vi "Decimate.vi"() -> (3 "2-Stage Decimation: Octaves 2-8":T1[](array[typedef])=[{"VSignalRMS"=3.569254560184283, "VNoiseRMS"=0.0015456498604675313, "SNR(dB)"=67.26932808076202, "NumBits"=10.881948186173094, "SNRFS(dB)"=67.18687774967906, "NumBitsFS"=10.868252117886886}, {"VSignalRMS"=3.569302135994948, "VNoiseRMS"=0.0015758831325008, "SNR(dB)"=67.1011860962303, "NumBits"=10.854017623958521, "SNRFS(dB)"=67.01861998873524, "NumBitsFS"=10.840302323710173}, {"VSignalRMS"=3.569179527030871, "VNoiseRMS"=0.0015457687304173328, "SNR(dB)"=67.26847751090318, "NumBits"=10.881806895498867, "SNRFS(dB)"=67.18620977720272, "NumBitsFS"=10.868141159003773}, {"VSignalRMS"=3.569284052806068, "VNoiseRMS"=0.0015488080787911924, "SNR(dB)"=67.25167012588723, "NumBits"=10.879014971077613, "SNRFS(dB)"=67.16914802390777, "NumBitsFS"=10.865306980715575}, {"VSignalRMS"=3.569278212241904, "VNoiseRMS"=0.0015445316735475394, "SNR(dB)"=67.27567164377996, "NumBits"=10.883001934182717, "SNRFS(dB)"=67.1931637548854, "NumBitsFS"=10.86929630479824}, {"VSignalRMS"=3.5692565348659597, "VNoiseRMS"=0.0010534504316992595, "SNR(dB)"=70.59927315773149, "NumBits"=11.435095208925496, "SNRFS(dB)"=70.51681802120187, "NumBitsFS"=11.421398342392337}, {"VSignalRMS"=3.569299509403375, "VNoiseRMS"=0.0007252888840803322, "SNR(dB)"=73.84143941716077, "NumBits"=11.97366103275096, "SNRFS(dB)"=73.75887970147343, "NumBitsFS"=11.95994679426469}, {"VSignalRMS"=3.569262170230891, "VNoiseRMS"=0.0004828117383160924, "SNR(dB)"=77.3760125744556, "NumBits"=12.560799430972692, "SNRFS(dB)"=77.29354372411225, "NumBitsFS"=12.547100286397384}, {"VSignalRMS"=3.56927087447335, "VNoiseRMS"=0.00037148318496641716, "SNR(dB)"=79.65280695478424, "NumBits"=12.93900447753891, "SNRFS(dB)"=79.57031692247287, "NumBitsFS"=12.925301814364264}] {"SNRFS(dB)" format="%_3p"; "NumBitsFS" format="%.1f"; "NumBits" format="%.1f"; "SNR(dB)" format="%_3p"; "VNoiseRMS" format="%#_3p"; "VSignalRMS" format="%#_3p"}, 11 "Input":waveform(dbl)[](graph)=[{"t0"=timestamp(0 s since 1904-01-01), "dt"=1e-07, "Y"=array[200000 elements]}, {"t0"=timestamp(0 s since 1904-01-01), "dt"=1e-07, "Y"=array[200000 elements]}] caption="Histogram")   [LabVIEW 2019] (continued)
-89.8010347026674, -91.03397353010905, -93.05880817130885, -93.86569223660774, -93.37353857073721, -94.99416885665839, -99.05596611693173, -107.36497646738917, -102.6044915270977, -96.19397229786782, -96.1597538289888, -102.83527542224925, -97.10995031748254, -93.13768460557588, -93.6872108649518, -96.88332215210443, -91.8911442399971, -88.87814381179629, -89.52765316051676, -90.61283401268693, -88.61347146837466, -86.64246320759895, -87.20248076787445, -89.71664016321188, -92.17437436351524, -96.52818073700101, -102.89028350758038, -95.51571015309541, -90.29404249884288, -88.78950020057246, -90.05141478281257, -93.14256393856814, -96.4338383803238, -98.1272334355839, -98.38148782151309, -98.52874806510161, -97.52896129220633, -93.04723881975156, -88.27184928640632, -85.88377796724602, -85.65268972364586, -86.59982678770758, -88.4789647414978, -91.7805915661704, -97.07047803294813, -107.73747761660528, -98.60351784227328, -93.52998614692484, -93.33290182993952, -96.85531600078095, -96.37376134080165, -90.69117698738063, -88.14576852093532, -88.25747447952166, -90.45082399151303, -96.41863707301175, -101.4196021122521, -93.96770566579788, -93.58811415156053, -96.07316515859912, -95.5343037432213, -96.69546499020845, -103.82710137540842, -91.0904529950192, -86.73242770513536, -86.46505143994031, -88.73991396184971, -92.4473353636468, -95.59367731654704, -91.48494027019697, -87.58229561240861, -85.91683271877996, -85.80490261027448, -86.60468865692945, -88.2671187787114, -91.43151609166779, -96.08162874738761, -97.96724691276759, -97.11638853174621, -99.15289822897408, -123.93308240573889, -100.23264801665928, -97.93670882000998, -101.99411747199824, -108.2661715906857, -95.01879672304669, -93.09344762172648, -97.96569428999419, -103.31348133169591, -94.56331004427977, -91.27392525391764, -89.86929621291289, -90.5326639141475, -93.30981422202001, -94.64433988957715, -93.81030718221622, -92.11600765997169, -90.47514602466164, -91.6034286338698, -91.52808955554679, -88.72387392453297, -90.22769969249696, -101.22756810629461, -93.02935870824089, -88.75723657607486, -89.07116344980949, -91.5022695405016, -92.33189422244578, -92.15231627049769, -96.429614181429, -97.34230671596741, -90.58396100985783, -87.14766416331051, -85.85891058335328, -86.31876359404814, -89.10677082541883, -97.31293864995898, -101.61260941340501, -96.67024962948099, -95.7803144954672, -92.23018395709333, -91.92293467829664, -95.19175145715253, -100.08921092086965, -100.05799390116158, -99.02803629195597, -109.28207521152451, -96.6021839187509, -90.38957395013965, -90.28504566646042, -93.17850262164265, -93.71200868183445, -97.4244039887505, -97.21740806348627, -89.14256467259328, -87.44588011755873, -90.97086244268247, -109.87431813081962, -96.94460754937701, -93.86113811879602, -91.86280043107433, -91.70994113858619, -92.89616081483194, -90.50118183916814, -90.18614880163818, -94.52151436094952, -100.73253124580648, -99.8220360349123, -100.29830396810995, -107.49078067194083, -94.01601739016263, -91.24863884043859, -94.98674357343711, -104.57651242950692, -99.85629224470014, -108.93064387422969, -93.53962952692434, -90.00240167674333, -90.68494946709862, -93.29637143102863, -94.60776650516321, -92.67968715579968, -90.33204021940706, -90.55631207399716, -92.43577805509032, -89.15503146181992, -86.30010955844271, -86.83979289314496, -89.48485493821893, -88.96405338383319, -87.52421931179818, -87.60531529349264, -88.6702529441048, -90.89292417707969, -95.88440563526038, -96.46881508553417, -91.06541812352924, -91.35314766368683, -99.08109799743801, -93.35876385631522, -88.11981688709662, -86.17097485203567, -85.52792069986612, -86.04182686687071, -88.51643246854445, -95.16445751359271, -100.73666271200408, -92.65818704084369, -93.12039396890881, -101.9336312438025, -96.2875533856691, -92.86539060044441, -92.38339167479018, -91.61776239409015, -89.00733167601517, -86.75068814616338, -86.11927241760986, -86.43308873694038, -86.39221303948099, -86.66783030203213, -88.67265978744017, -92.24294564543717, -95.12190286714484, -95.27152864373058, -93.34130562149033, -89.80175424374963, -87.41382180737244, -88.04182405274452, -91.15829518615249, -94.8596085864744, -99.07780397052106, -95.01095310320474, -91.45492540453984, -88.85659471003605, -88.09703705871516, -91.14850708600869, -102.48113857609522, -95.20951614488438, -90.76054140267786, -89.82778110342488, -90.66593638186606, -91.75679507239694, -90.08765062811106, -88.65512843108004, -89.86771840104606, -93.11899129528413, -95.07880434483995, -93.66805564380138, -91.82378563741104, -91.42798403486283, -93.33242715271743, -94.46541343567961, -95.10490793802889, -95.23778068069765, -89.91147243285879, -84.72844146564022, -83.12294491520029, -84.9529908072355, -89.20201404077906, -93.39646902993033, -90.84293632205467, -88.26483479024421, -87.52146927444474, -88.27666880088361, -89.15187738597957, -90.11954936247787, -94.16844824268043, -107.89828675933434, -92.96950334185829, -88.238044809099, -86.53155469309384, -86.00724711483737, -85.84166713830888, -86.34560567244318, -88.05752912180658, -89.45912806461533, -89.2035558192775, -90.26794762923997, -94.61492559085042, -93.47913197993867, -89.68023195055093, -88.5844007239764, -88.16209645670403, -87.69248229261242, -88.19926215150255, -89.03813165364234, -88.23806114711809, -86.06271848210922, -84.55338844577818, -84.60581192467787, -85.1077884922066, -84.87483822256023, -86.29645607493103, -92.06433822589182, -107.45719303754848, -112.34185245802342, -100.81236537855537, -95.98023535529101, -97.06022523776083, -108.91939984092842, -104.58355826222842, -105.28926347697224, -98.10962881250319, -91.97176200903287, -90.1266388214861, -90.67818031849367, -92.85563489938073, -93.76500929039366, -91.5852495688892, -91.19048588685934, -93.62384628504867, -93.7795356927555, -91.19750841744859, -90.74358943616139, -93.00542929634658, -94.3681235267732, -90.8623272907447, -90.01485035029057, -92.52070202183269, -98.91906043598311, -102.5897642561925, -99.82530029415895, -102.20958845474463, -107.13921947376252, -107.01853509868056, -110.28556884145588, -103.44422077868307, -94.7252960700585, -91.45806458223853, -93.42525832838932, -97.31725729774752, -95.44946115186846, -94.8595760042268, -94.1498831531218, -93.04365469327082, -92.03054869023626, -91.77414183713913, -94.41138276683348, -98.48171674510718, -95.05341322220156, -94.82148351748654, -97.08324798828943, -92.96605208041271, -89.34070749513245, -88.29777010929871, -88.30288027606483, -89.48962380854178, -93.82108906158335, -96.51961583222484, -95.21010881511009, -100.42640215279664, -108.00389623621597, -100.31346689277512, -98.771133498524, -96.92097352108053, -96.52772982975304, -103.85461800825347, -98.4364859896675, -96.75691862450641, -99.93868436121357, -101.0553868817555, -101.80612831811997, -102.32522849853484, -114.90329875071347, -97.84170076615057, -90.72356335005702, -88.75686077967089, -90.93220347773621, -100.31068639097393, -92.6918740853231, -87.47727509271918, -86.40638848521573, -87.31674769566013, -88.8718261906175, -90.84717782219451, -96.14111518295532, -112.7387467405839, -96.80330128832384, -94.49443144832229, -93.1187694720117, -94.09577295380575, -97.84347233566405, -98.83196403782361, -102.66702576290031, -102.06740338682923, -96.98779181032735, -95.60219419087134, -96.27567410728503, -97.38558620235028, -101.70178505678969, -105.17955779424086, -92.53192910654218, -88.81788220476069, -88.95711618627857, -92.57722780091505, -95.93532470547275, -94.91138856116832, -94.10808424076805, -91.07784296453154, -90.66312583820053, -94.83055022969745, -93.45801693898999, -88.36453147845204, -86.51183079184831, -86.25944696127009, -87.45497047294643, -89.96042118208382, -92.69280919745722, -95.17516080722282, -97.2545095704103, -108.19727080658595, -94.98874557277178, -88.7096850874034, -88.29851760651509, -92.97093470402908, -109.47313678444067, -92.15693004585063, -89.54380160860075, -91.20532066404374, -94.01507769477956, -98.32922344795767, -115.87223636278607, -104.99730428404263, -97.90500783504449, -93.52723553984637, -92.68564560569936, -95.29601374056632, -98.60820212308043, -95.8632487136141, -95.62504147674952, -96.80363703429067, -93.03623657868951, -90.52579360619532, -90.264401776805, -92.92037685812984, -103.55931238637702, -100.10371390759235, -97.64269926597996, -106.70160125220791, -103.46147653543306, -104.92381444474447, -97.66898940024639, -98.1207217224727, -102.97619867092016, -98.71215110846583, -97.0432854793485, -99.16590358458605, -108.7063174536745, -100.82749343291766, -96.03893851051149, -91.58971668752456, -89.61426914396401, -90.35560864138453, -92.20810749474501, -92.89100216232576, -93.49681684033557, -99.76551973814325, -97.0799906106162, -90.31362726389034, -88.57325340330499, -88.96730438665082, -90.26248640164394, -90.52895855114714, -90.20987348700926, -93.00267887063752, -94.17584736186727, -88.81040704570617, -86.93952112623633, -87.9056288932579, -91.98566538263984, -100.15858921606016, -103.76052918019197, -96.71723266703998, -93.03577725134335, -94.72780454891021, -103.01451117711142, -97.6699107089091, -96.01913455617363, -110.1206312200923, -91.92605804348743, -88.00078024686586, -87.8880681034834, -87.30056231006418, -85.83303495316628, -85.85418846348472, -87.7821464251187, -90.2758402998394, -90.88533878280161, -90.8459208229611, -93.28890303633764, -96.45506943175144, -93.9657279319056, -95.14678514742427, -103.76092783519839, -93.51369734169444, -89.15496358093812, -88.94760221872505, -93.21836724942621, -102.70177680497022, -94.3088663314495, -94.4492283335647, -107.54669077263702, -95.02325691171124, -89.94809305281855, -88.76442278570764, -90.15843384117183, -94.18927428924788, -103.5607343640872, -104.71985453910293, -97.44689724688605, -96.66538549864534, -92.99791884731977, -88.91345920971567, -88.78289126806351, -93.20237581867212, -99.61032143489241, -98.03939989557719, -93.0026775167182, -91.81883719675187, -93.16528083057023, -91.99657831882547, -90.82862397733015, -90.35913544748666, -88.27997681101144, -87.06043651234096, -90.01623158825575, -98.26998906374854, -98.87182053703206, -97.96821523251893, -100.72261242087296, -103.61735109062678, -100.97137969331385, -96.99686450208753, -99.11583654269441, -96.80933076136141, -89.94358046453371, -90.5589653328009, -98.05169889385459, -93.71424181113524, -90.43633068673337, -92.57816106624148, -103.50808505873314, -100.01204811846273, -93.81345468138845, -92.31007899066856, -92.41740595409402, -92.79570377679568, -93.82486981119445, -98.31226033178805, -101.74612278185292, -94.3497825868709, -90.69857292290774, -88.78277526094769, -88.77097805601, -89.94284365081724, -90.70689274098581, -91.5148685235682, -93.14799332791, -94.81640407745275, -98.81943039379316, -106.08095876700384, -95.18999798662253, -92.4142146852307, -92.57021663897197, -92.66199047832845, -91.92099703946455, -90.03706209531208, -87.38587815679551, -85.87225930549337, -86.2255296819672, -88.28775142723944, -93.27505872274777, -115.99751912628982, -92.53915821293742, -87.9207035231365, -85.55641230589154, -84.94877133314154, -86.88955282712729, -93.96785309236557, -94.0289793243198, -87.4272553612049, -87.29762396991052, -92.30440971489529, -120.21878514409582, -95.00976512147977, -91.31588049120478, -90.56898331734459, -90.77858748375854, -91.89648836362517, -96.29348753218406, -100.93249278623325, -97.32178285939624, -98.62014208276622, -100.48562472201668, -97.33369690760833, -95.00343910264645, -95.69979646246864, -98.74130162362789, -100.27898936972626, -94.9378052586386, -90.20931572958756, -88.53058670603681, -88.27380374992417, -87.20092602666031, -86.05931266172865, -87.22653057818638, -91.39673283963971, -95.38223908175, -95.96072073705783, -99.42329566628243, -98.34654372546375, -93.4993314587484, -92.89016890488827, -92.02184448181553, -92.17619172419795, -96.26933765840184, -98.18453485909882, -93.66052810216247, -90.8323686849731, -90.36431799650393, -91.97615119961696, -96.46500758909855, -94.96914243908718, -91.01807463861238, -91.2779918513813, -92.96017533514774, -95.42849867438704, -101.77004213826638, -105.27901395308567, -99.56242545898206, -97.90225814801475, -101.28031650242258, -96.1015978589149, -93.34246627165528, -93.70559141177273, -94.20889705360737, -93.81582595663994, -94.06324580025588, -95.19473180113226, -92.86573512497009, -89.18354883248035, -88.20359411470437, -89.89806767859326, -91.91816476953262, -89.77231066774974, -88.18071979990691, -88.0280893835839, -88.04423231379133, -88.80392977533683, -91.19824097961524, -98.58922742068387, -95.30068248468645, -90.02940744460808, -89.92923732451595, -96.44564808729093, -99.96939540191892, -91.78821600214482, -91.34013881425585, -91.68182786268892, -92.75576407614253, -97.60096039215023, -110.79584639656908, -100.7398169767965, -98.90169971973356, -96.98475068395564, -91.24777218925851, -87.14164582650936, -85.07841513945877, -85.26972079412609, -87.22392671417005, -88.00822550141241, -87.76027181453824, -89.58415902951826, -92.4920968244888, -91.52877820490346, -90.95171438597555, -95.41394558528829, -107.52016977965116, -93.55378221755299, -93.09841424146704, -96.03020240280674, -92.62019862066694, -90.37102864174886, -90.32746097852643, -91.64498883121686, -90.32100090650229, -87.3315532070872, -85.03676944258837, -83.85985926521577, -84.73848912491917, -87.6784018437611, -90.04115270468093, -91.25387893030472, -93.23095692661319, -95.25231864597927, -97.66363332944596, -102.77464914802627, -101.15895720449821, -99.62005914650605, -102.63735241934043, -104.85039530539925, -101.25579402001435, -99.77764723417644, -101.57938969988805, -99.1058053458501, -96.33289113064549, -94.41799875122697, -93.49242925347608, -94.50404330381863, -96.76817317436303, -93.93672457673864, -91.29474684489637, -93.26842869447049, -102.42081187230232, -103.08983670436645, -109.52250784041115, -97.2726279572302, -89.96149106309333, -88.13167591404391, -89.17627713478488, -90.81731028389734, -89.69598642936998, -89.38981783502201, -89.50603404532913, -88.89585545757966, -89.56629637073901, -90.96578900098268, -91.22149297466228, -91.3785919844561, -93.15397967041592, -94.4901683525819, -92.7368020668827, -92.14949353336037, -94.95758584517533, -103.64001941535494, -102.27201854610108, -94.06232889812578, -92.93522322915264, -95.7335577608483, -97.6724118748942, -93.40509883173105, -93.66687115451643, -101.02764174706243, -99.12707487021106, -94.48016277568419, -94.67470865634454, -98.42431273446714, -103.24880029559685, -99.90925994581126, -95.15695525887934, -93.41579558721341, -94.67409325043697, -95.82278490747215, -94.14142963683659, -93.06397710154005, -94.67664396404518, -98.33033807601927, -93.38609170228307, -90.11276515968119, -88.90838552954386, -87.56195891881562, -86.61620485564832, -87.44524687073933, -90.90537825376526, -96.54713542070294, -93.39343846176016, -91.65569563103823, -92.14374689709948, -93.25103368600128, -97.10001809735326, -92.95120769052104, -86.90162204337808, -85.96113002826127, -89.22843563290024, -99.98215601142925, -93.87545654951096, -88.52698412964402, -90.35913274669417, -100.91895124333183, -92.48828884459081, -89.52817506852307, -90.85947850957027, -94.57527777304777, -99.5269326990987, -99.60633181869059, -95.72628145429307, -95.03394942536164, -94.1117243729267, -92.45824814083, -93.20733286443966, -94.21187595555205, -91.14499167368595, -88.47301855464184, -87.65697415447646, -89.3491095696534, -93.80345111261569, -99.68008971154478, -100.12908406450812, -94.31594799973227, -92.32494145325448, -93.75927524111154, -93.24162555187677, -91.83340564056253, -91.39583615477781, -92.9927938979383, -99.32988111167916, -102.36851511008263, -94.21226623786877, -89.50102510569984, -87.52005746489233, -88.47429326228288, -94.18062027460594, -97.08519622981159, -88.44622877710566, -87.17483083286665, -90.53412682553531, -98.80032159988284, -112.0139605538499, -114.73822729493698, -108.47097394029929, -107.04801965347384, -103.79117249163477, -93.69620484132517, -90.20414443914342, -90.93394829658737, -93.89847212895639, -95.25161152513147, -94.67463116505695, -94.65303698780667, -96.52871287518005, -103.59167379262703, -97.3093661652524, -93.13057204576113, -93.48726944940366, -96.97938502988173, -100.05124973201501, -94.39188624348108, -91.47606085909311, -92.9112596329322, -96.52898769576653, -95.93029258632751, -91.36739129728717, -90.64709732022601, -92.33074646702256, -93.12266929064732, -92.710435012283, -93.66993194171718, -96.66266310132755, -101.86758330767772, -102.0049247869093, -97.6442479953907, -95.68999770184644, -95.70255601030347, -91.85350103951814, -88.66409645137753, -88.97899246700999, -92.47972679191342, -94.19740594455185, -89.79975447682834, -88.06347092046212, -89.50744525042023, -94.90319594188456, -102.73396352972853, -97.78022699866135, -96.41875055142742, -97.61374856205884, -101.14594314754896, -91.07819652365637, -86.20151492090294, -84.43580987646789, -84.40343321539262, -85.4512275674312, -86.95812160502341, -87.38158628291737, -86.92750011319069, -87.59641317432796, -90.8808100008769, -98.66278213466741, -92.07358739303535, -86.66872385575152, -84.81103040399233, -85.15216430890109, -86.3701227119982, -86.99273267548816, -87.56139630381969, -89.59164806271204, -93.90931125716035, -94.7747826643407, -90.81810446669623, -88.25377581259738, -86.89687153931219, -87.00420294319926, -89.66919632785404, -97.97802217885085, -101.1543714645282, -92.01004343018782, -88.48812761828798, -86.37140706971644, -85.30861499609067, -85.50676823397659, -87.04715207432281, -89.56919372991476, -91.21639006182731, -90.00710468462273, -87.56326618667731, -85.71087905629356, -85.256302358152, -86.02039260583963, -85.95860793013176, -84.9597151895099, -85.47467902194902, -88.17529871401237, -94.46151142269389, -104.4795994742826, -90.62205386572919, -86.60259576725531, -86.15117934101244, -88.14061646864911, -90.22552942827053, -90.23075884569806, -88.9795464994569, -88.09496890634763, -88.10286347397336, -89.29342654721987, -91.97001454391268, -94.97369664752816, -94.58282592742778, -93.03651295821604, -91.73180808496429, -89.4413987639919, -88.1062492362812, -89.08416681250316, -92.00463005101325, -94.46986101023663, -94.98934726061613, -94.75619871742677, -95.15939521180876, -100.30338510222867, -100.72723563767974, -90.65610684683526, -87.78121672994476, -88.9486698831994, -94.27478448469651, -103.54935817879945, -98.06669656253065, -93.91758818564313, -93.47079131141024, -92.04208725685709, -90.6451361739226, -90.76636107274352, -90.42103213618275, -90.56286879665706, -91.72390699440554, -94.00932025463854, -101.33128658211626, -105.61432288405747, -100.71871174366068, -95.43418166984756, -91.226388311365, -92.05115080560162, -94.90602236858494, -94.7278081014079, -92.50147105725247, -91.73088417004178, -93.99995298481683, -100.77630752561265, -92.24736653451953, -87.34945508143532, -86.32547617096144, -87.72396565284308, -91.61940201299744, -102.83952571655541, -98.57454225038964, -92.11235735605948, -90.82153081888086, -93.22653255311293, -100.57820257707947, -100.71490844146241, -93.27806436638666, -89.81672883858188, -89.43584378033519, -91.49478107995014, -91.23005227675968, -89.87906075424215, -91.22224554955343, -94.36330957997907, -96.57020876047248, -98.47960211136326, -102.60206932430148, -97.85025869384859, -95.62004803407247, -96.82074626938368, -95.36641190186579, -94.62955480252799, -96.56732905283187, -99.78488099782834, -95.54134836047314, -90.85106276396188, -91.53811864957345, -97.35398945483547, -99.53390924269618, -95.50550211172002, -94.24883407244174, -95.15845296283891, -92.52876949052072, -89.18489265592221, -88.3231593450649, -90.21847755944741, -96.28601451043076, -96.42148418004156, -90.0423710177557, -88.35384430411479, -88.45800104614098, -87.39915267866814, -84.9649415862749, -83.05546796952149, -82.53813288647429, -83.62358980677735, -86.64329516486029, -92.49839132920357, -100.96627720063958, -102.03774536659961, -101.55721936960227, -101.4919591633547, -109.49368516118811, -100.54156324375568, -93.1995924271338, -91.95610626225269, -94.54326224475864, -94.45480287553445, -90.63645329465285, -89.06115591026294, -89.13290400541244, -89.03992767460898, -88.35162930135266, -88.46227802743762, -88.71864528174883, -87.14494782239026, -85.75618719388423, -86.7517555817581, -89.70602126044467, -91.9312021642449, -93.10715040857424, -95.09804072655095, -93.67107590708542, -88.79809377890399, -85.4813978604545, -84.97790290229165, -87.26875120136336, -91.81955749355437, -93.97436752534212, -93.17419492057974, -94.72899092677758, -101.50873916930624, -102.42854835344474, -90.93542725599947, -86.91428707756133, -87.10383889824635, -89.09108940684278, -88.4500883642402, -86.62101390069743, -85.92383744773456, -85.91510889390906, -85.89392970945173, -86.18538075642498, -87.06255280982421, -89.6041373377338, -97.37862658290312, -96.5067648178377, -89.45694870912129, -86.72282125077987, -84.7805642597111, -82.9102759515595, -82.19689500929915, -83.06278673741679, -84.61305596458077, -85.57445584067696, -86.0152215595378, -86.49448845038934, -86.21839866020926, -85.33030186000204, -86.20000801703499, -90.11626361376807, -93.71043548054743, -91.20571923212147, -88.34768634049867, -88.05561567210353, -90.11882678795826, -92.79075903663114, -92.53274818890827, -90.15586226108351, -89.7588785406825, -92.51437122484617, -96.88253109308307, -95.01965867485444, -89.4020940322562, -87.36029269867059, -88.40574804749141, -89.39108945249801, -89.2136953159512, -90.0825705642915, -93.5797629864681, -100.02421686821893, -97.37689573314105, -91.15170800268984, -89.62276780794588, -91.81358650078799, -96.1459571696283, -98.78905079920406, -95.90966812857447, -91.0005558312157, -89.42715635616975, -91.23884179011795, -97.4530564846785, -103.85666825119125, -96.25176115537727, -93.62539913970993, -93.03047254411906, -93.6940820406606, -93.61728990851228, -90.37925780092463, -87.38864297445694, -88.18397636144071, -96.3132450903164, -89.02089079629584, -84.41432793280624, -83.65030393991381, -84.44637248702462, -85.87910745894929, -87.96238438851253, -90.95552843255147, -95.23385561565782, -99.98676571010093, -98.25033889671077, -92.9148387998585, -90.76261672348406, -92.44105364838288, -97.36071315590407, -102.36442424446955, -106.64846134350339, -100.6227402487165, -96.18879414360443, -94.50781769211488, -94.24616329879782, -93.08870297958529, -93.04485425173121, -97.00614950521859]} caption="Histogram"
  out "filter information 2":T3={"magnitude H(w)"={"f0"=0.0, "df"=4882.8125, "Mag H(w)"=[0.0, 0.0, 0.0, -0.0, 0.0, 0.0, -0.0, -0.0, -0.0, 0.0, 0.0, 0.0, 0.0, 0.0, 0.0, 0.0, 0.0, -0.0, -0.0, -0.0, -0.0, -0.0, -0.0, -0.0, -0.0, -0.0, -0.0, -0.0, -0.0, -0.0, -0.0, -0.0, 0.0, 0.0, 0.0, 0.0, 0.0, 0.0, 0.0, 0.0, 0.0, 0.0, 0.0, 0.0, 0.0, 0.0, 0.0, 0.0, 0.0, -0.0, -0.0, -0.0, -0.0, -0.0, -0.0, -0.0, -0.0, -0.0, -0.0, -0.0, -0.0, -0.0, -0.0, -0.0, 0.0, 0.0, 0.0, 0.0, 0.0, 0.0, 0.0, 0.0, 0.0, 0.0, 0.0, 0.0, 0.0, 0.0, 0.0, 0.0, 0.0, -0.0, -0.0, -0.0, -0.0, -0.0, -0.0, -0.0, -0.0, -0.0, -0.0, -0.0, -0.0, -0.0, -0.0, -0.0, -0.0, 0.0, 0.0, 0.0, 0.0, 0.0, 0.0, 0.0, 0.0, 0.0, 0.0, 0.0, 0.0, 0.0, 0.0, 0.0, 0.0, -0.0, -0.0, -0.0, -0.0, -0.0, -0.0, -0.0, -0.0, -0.0, -0.0, -0.0, -0.0, -0.0, -0.0, -0.0, 0.0, 0.0, 0.0, 0.0, 0.0, 0.0, 0.0, 0.0, 0.0, 0.0, 0.0, 0.0, 0.0, 0.0, 0.0, 0.0, 0.0, -0.0, -0.0, -0.0, -0.0, -0.0, -0.0, -0.0, -0.0, -0.0, -0.0, -0.0, -0.0, -0.0, -0.0, -0.0, 0.0, 0.0, 0.0, 0.0, 0.0, 0.0, 0.0, 0.0, 0.0, 0.0, 0.0, 0.0, 0.0, 0.0, 0.0, 0.0, 0.0, -0.0, -0.0, -0.0, -0.0, -0.0, -0.0, -0.0, -0.0, -0.0, -0.0, -0.0, -0.0, -0.0, -0.0, -0.0, -0.0, 0.0, 0.0, 0.0, 0.0, 0.0, 0.0, 0.0, 0.0, 0.0, 0.0, 0.0, 0.0, 0.0, 0.0, 0.0, 0.0, -0.0, -0.0, -0.0, -0.0, -0.0, -0.0, -0.0, -0.0, -0.0, -0.0, -0.0, -0.0, -0.0, -0.0, -0.0, -0.0, 0.0, 0.0, 0.0, 0.0, 0.0, 0.0, 0.0, 0.0, 0.0, 0.0, 0.0, 0.0, 0.0, 0.0, 0.0, 0.0, -0.0, -0.0, -0.0, -0.0, -0.0, -0.0, -0.0, -0.0, -0.0, -0.0, -0.0, -0.0, -0.0, -0.0, -0.0, -0.0, 0.0, 0.0, 0.0, 0.0, 0.0, 0.0, 0.0, 0.0, 0.0, 0.0, 0.0, 0.0, 0.0, 0.0, 0.0, 0.0, -0.0, -0.0, -0.0, -0.0, -0.0, -0.0, -0.0, -0.0, -0.0, -0.0, -0.0, -0.0, -0.0, -0.0, -0.0, 0.0, 0.0, 0.0, 0.0, 0.0, 0.0, 0.0, 0.0, 0.0, 0.0, 0.0, 0.0, 0.0, 0.0, 0.0, 0.0, 0.0, -0.0, -0.0, -0.0, -0.0, -0.0, -0.0, -0.0, -0.0, -0.0, -0.0, -0.0, -0.0, -0.0, -0.0, -0.0, 0.0, 0.0, 0.0, 0.0, 0.0, 0.0, 0.0, 0.0, 0.0, 0.0, 0.0, 0.0, 0.0, 0.0, 0.0, 0.0, 0.0, -0.0, -0.0, -0.0, -0.0, -0.0, -0.0, -0.0, -0.0, -0.0, -0.0, -0.0, -0.0, -0.0, -0.0, -0.0, 0.0, 0.0, 0.0, 0.0, 0.0, 0.0, 0.0, 0.0, 0.0, 0.0, 0.0, 0.0, 0.0, 0.0, 0.0, 0.0, 0.0, -0.0, -0.0, -0.0, -0.0, -0.0, -0.0, -0.0, -0.0, -0.0, -0.0, -0.0, -0.0, -0.0, -0.0, -0.0, 0.0, 0.0, 0.0, 0.0, 0.0, 0.0, 0.0, 0.0, 0.0, 0.0, 0.0, 0.0, 0.0, 0.0, 0.0, 0.0, 0.0, -0.0, -0.0, -0.0, -0.0, -0.0, -0.0, -0.0, -0.0, -0.0, -0.0, -0.0, -0.0, -0.0, -0.0, -0.0, 0.0, 0.0, 0.0, 0.0, 0.0, 0.0, 0.0, 0.0, 0.0, 0.0, 0.0, 0.0, 0.0, 0.0, 0.0, 0.0, 0.0, -0.0, -0.0, -0.0, -0.0, -0.0, -0.0, -0.0, -0.0, -0.0, -0.0, -0.0, -0.0, -0.0, -0.0, -0.0, 0.0, 0.0, 0.0, 0.0, 0.0, 0.0, 0.0, 0.0, 0.0, 0.0, 0.0, 0.0, 0.0, 0.0, 0.0, 0.0, 0.0, -0.0, -0.0, -0.0, -0.0, -0.0, -0.0, -0.0, -0.0, -0.0, -0.0, -0.0, -0.0, -0.0, -0.0, -0.0, 0.0, 0.0, 0.0, 0.0, 0.0, 0.0, 0.0, 0.0, 0.0, 0.0, 0.0, 0.0, 0.0, 0.0, 0.0, 0.0, 0.0, -0.0, -0.0, -0.0, -0.0, -0.0, -0.0, -0.0, -0.0, -0.0, -0.0, -0.0, -0.0, -0.0, -0.0, -0.0, 0.0]}, "phase H(w)"={"f0"=0.0, "df"=4882.8125, "Phase H(w)"=[0.0, 0.0, 0.0, -0.0, 0.0, 0.0, -0.0, -0.0, -0.0, 0.0, 0.0, 0.0, 0.0, 0.0, 0.0, 0.0, 0.0, -0.0, -0.0, -0.0, -0.0, -0.0, -0.0, -0.0, -0.0, -0.0, -0.0, -0.0, -0.0, -0.0, -0.0, -0.0, 0.0, 0.0, 0.0, 0.0, 0.0, 0.0, 0.0, 0.0, 0.0, 0.0, 0.0, 0.0, 0.0, 0.0, 0.0, 0.0, 0.0, -0.0, -0.0, -0.0, -0.0, -0.0, -0.0, -0.0, -0.0, -0.0, -0.0, -0.0, -0.0, -0.0, -0.0, -0.0, 0.0, 0.0, 0.0, 0.0, 0.0, 0.0, 0.0, 0.0, 0.0, 0.0, 0.0, 0.0, 0.0, 0.0, 0.0, 0.0, 0.0, -0.0, -0.0, -0.0, -0.0, -0.0, -0.0, -0.0, -0.0, -0.0, -0.0, -0.0, -0.0, -0.0, -0.0, -0.0, -0.0, 0.0, 0.0, 0.0, 0.0, 0.0, 0.0, 0.0, 0.0, 0.0, 0.0, 0.0, 0.0, 0.0, 0.0, 0.0, 0.0, -0.0, -0.0, -0.0, -0.0, -0.0, -0.0, -0.0, -0.0, -0.0, -0.0, -0.0, -0.0, -0.0, -0.0, -0.0, 0.0, 0.0, 0.0, 0.0, 0.0, 0.0, 0.0, 0.0, 0.0, 0.0, 0.0, 0.0, 0.0, 0.0, 0.0, 0.0, 0.0, -0.0, -0.0, -0.0, -0.0, -0.0, -0.0, -0.0, -0.0, -0.0, -0.0, -0.0, -0.0, -0.0, -0.0, -0.0, 0.0, 0.0, 0.0, 0.0, 0.0, 0.0, 0.0, 0.0, 0.0, 0.0, 0.0, 0.0, 0.0, 0.0, 0.0, 0.0, 0.0, -0.0, -0.0, -0.0, -0.0, -0.0, -0.0, -0.0, -0.0, -0.0, -0.0, -0.0, -0.0, -0.0, -0.0, -0.0, -0.0, 0.0, 0.0, 0.0, 0.0, 0.0, 0.0, 0.0, 0.0, 0.0, 0.0, 0.0, 0.0, 0.0, 0.0, 0.0, 0.0, -0.0, -0.0, -0.0, -0.0, -0.0, -0.0, -0.0, -0.0, -0.0, -0.0, -0.0, -0.0, -0.0, -0.0, -0.0, -0.0, 0.0, 0.0, 0.0, 0.0, 0.0, 0.0, 0.0, 0.0, 0.0, 0.0, 0.0, 0.0, 0.0, 0.0, 0.0, 0.0, -0.0, -0.0, -0.0, -0.0, -0.0, -0.0, -0.0, -0.0, -0.0, -0.0, -0.0, -0.0, -0.0, -0.0, -0.0, -0.0, 0.0, 0.0, 0.0, 0.0, 0.0, 0.0, 0.0, 0.0, 0.0, 0.0, 0.0, 0.0, 0.0, 0.0, 0.0, 0.0, -0.0, -0.0, -0.0, -0.0, -0.0, -0.0, -0.0, -0.0, -0.0, -0.0, -0.0, -0.0, -0.0, -0.0, -0.0, 0.0, 0.0, 0.0, 0.0, 0.0, 0.0, 0.0, 0.0, 0.0, 0.0, 0.0, 0.0, 0.0, 0.0, 0.0, 0.0, 0.0, -0.0, -0.0, -0.0, -0.0, -0.0, -0.0, -0.0, -0.0, -0.0, -0.0, -0.0, -0.0, -0.0, -0.0, -0.0, 0.0, 0.0, 0.0, 0.0, 0.0, 0.0, 0.0, 0.0, 0.0, 0.0, 0.0, 0.0, 0.0, 0.0, 0.0, 0.0, 0.0, -0.0, -0.0, -0.0, -0.0, -0.0, -0.0, -0.0, -0.0, -0.0, -0.0, -0.0, -0.0, -0.0, -0.0, -0.0, 0.0, 0.0, 0.0, 0.0, 0.0, 0.0, 0.0, 0.0, 0.0, 0.0, 0.0, 0.0, 0.0, 0.0, 0.0, 0.0, 0.0, -0.0, -0.0, -0.0, -0.0, -0.0, -0.0, -0.0, -0.0, -0.0, -0.0, -0.0, -0.0, -0.0, -0.0, -0.0, 0.0, 0.0, 0.0, 0.0, 0.0, 0.0, 0.0, 0.0, 0.0, 0.0, 0.0, 0.0, 0.0, 0.0, 0.0, 0.0, 0.0, -0.0, -0.0, -0.0, -0.0, -0.0, -0.0, -0.0, -0.0, -0.0, -0.0, -0.0, -0.0, -0.0, -0.0, -0.0, 0.0, 0.0, 0.0, 0.0, 0.0, 0.0, 0.0, 0.0, 0.0, 0.0, 0.0, 0.0, 0.0, 0.0, 0.0, 0.0, 0.0, -0.0, -0.0, -0.0, -0.0, -0.0, -0.0, -0.0, -0.0, -0.0, -0.0, -0.0, -0.0, -0.0, -0.0, -0.0, 0.0, 0.0, 0.0, 0.0, 0.0, 0.0, 0.0, 0.0, 0.0, 0.0, 0.0, 0.0, 0.0, 0.0, 0.0, 0.0, 0.0, -0.0, -0.0, -0.0, -0.0, -0.0, -0.0, -0.0, -0.0, -0.0, -0.0, -0.0, -0.0, -0.0, -0.0, -0.0, 0.0, 0.0, 0.0, 0.0, 0.0, 0.0, 0.0, 0.0, 0.0, 0.0, 0.0, 0.0, 0.0, 0.0, 0.0, 0.0, 0.0, -0.0, -0.0, -0.0, -0.0, -0.0, -0.0, -0.0, -0.0, -0.0, -0.0, -0.0, -0.0, -0.0, -0.0, -0.0, 0.0]}, "order"=-1} {"phase H(w)"."df" format="%.2p"; "phase H(w)"."f0" format="%.2p"; "phase H(w)"."Phase H(w)" format="%.2p"; "magnitude H(w)"."df" format="%.2p"; "magnitude H(w)"."f0" format="%.2p"; "magnitude H(w)"."Mag H(w)" format="%.2p"}
  in  "optional FIR filter specifications 2":T4={"PB Gain"=0.086, "SB Gain"=-120.0, "Scale"=TRUE, "Window"=enum."None"} {"SB Gain" format="%.2p"; "PB Gain" format="%.2p"}
  out "filter information":T3={"magnitude H(w)"={"f0"=0.0, "df"=9765.625, "Mag H(w)"=array[513 elements]}, "phase H(w)"={"f0"=0.0, "df"=9765.625, "Phase H(w)"=array[513 elements]}, "order"=867} {"phase H(w)"."df" format="%.2p"; "phase H(w)"."f0" format="%.2p"; "phase H(w)"."Phase H(w)" format="%.2p"; "magnitude H(w)"."df" format="%.2p"; "magnitude H(w)"."f0" format="%.2p"; "magnitude H(w)"."Mag H(w)" format="%.2p"}
  in  "optional FIR filter specifications":T4={"PB Gain"=0.086, "SB Gain"=-120.0, "Scale"=TRUE, "Window"=enum."None"} {"SB Gain" format="%.2p"; "PB Gain" format="%.2p"}
  out "FIR filter specifications":T2={"Topology"=enum."FIR by Specification", "Type"=enum."Lowpass", "#Taps"=0, "Lower PB"=1200000.0, "Upper PB"=0.0, "Lower SB"=1250000.0, "Upper SB"=0.0} {"Lower SB" format="%0.2p"; "Upper SB" format="%0.2p"; "Lower PB" format="%0.2p"; "Upper PB" format="%0.2p"}
  in  "frequency 4":dbl=1001.0 format="%0.2p"
  in  "sampling info":cluster{"Fs":dbl, "#s":dbl}={"Fs"=10000000.0, "#s"=200000.0} {"Fs" format="%.2p"}
  in  "VRef 4":dbl=5.0
  in  "LowerNoiseBW":dbl
  in  "IgnoreDC":bool=TRUE
  out "delta 3":dbl=0.009765625
  out "QNoise (sigma)":dbl=0.00281909311127747
  out "2^(N-1)/Vref 3":dbl=102.4
  out "MeasSNRResults":T1={"VSignalRMS"=3.5355438607572442, "VNoiseRMS"=0.0015467583075278837, "SNR(dB)"=67.18067544121146, "NumBits"=10.867221834088284, "SNRFS(dB)"=67.18065098482452, "NumBitsFS"=10.867217771565535} {"SNRFS(dB)" format="%_3p"; "NumBitsFS" format="%.1f"; "NumBits" format="%.1f"; "SNR(dB)" format="%_3p"; "VNoiseRMS" format="%#_3p"; "VSignalRMS" format="%#_3p"}
  out "Mag Spectrum":cluster{"f0":dbl, "df":dbl, "magnitude":dbl[]}(graph)={"f0"=0.0, "df"=50.0, "magnitude"=array[100000 elements]} caption="Histogram"
  out "UpperNoiseBW":dbl=1250000.0
  out "Octave # (d)":i32=2
  out "2^d":dbl=4.0
  out "Results: Octaves 2-8":T1[](array[typedef])=[{"VSignalRMS"=3.535574020902194, "VNoiseRMS"=0.0022553181663702215, "SNR(dB)"=63.90504231916188, "NumBits"=10.323096730757788, "SNRFS(dB)"=63.904943767647424, "NumBitsFS"=10.323080360074323}, {"VSignalRMS"=3.535566614943483, "VNoiseRMS"=0.0015655999972608876, "SNR(dB)"=67.07556424946065, "NumBits"=10.849761503232667, "SNRFS(dB)"=67.07548389227816, "NumBitsFS"=10.849748154863482}, {"VSignalRMS"=3.5355406798310867, "VNoiseRMS"=0.0011061431804716454, "SNR(dB)"=70.09288984787959, "NumBits"=11.350978380046444, "SNRFS(dB)"=70.09287320618454, "NumBitsFS"=11.350975615645272}, {"VSignalRMS"=3.5355461411524223, "VNoiseRMS"=0.0007696216106961888, "SNR(dB)"=73.24358510813353, "NumBits"=11.874349685736467, "SNRFS(dB)"=73.24355504942477, "NumBitsFS"=11.874344692595477}, {"VSignalRMS"=3.535576343841796, "VNoiseRMS"=0.0005147833411276089, "SNR(dB)"=76.73671470273972, "NumBits"=12.454603771219222, "SNRFS(dB)"=76.73661044443189, "NumBitsFS"=12.454586452563436}, {"VSignalRMS"=3.5355527338895167, "VNoiseRMS"=0.00035740231649575695, "SNR(dB)"=79.90599912437312, "NumBits"=12.98106297747062, "SNRFS(dB)"=79.90595286909073, "NumBitsFS"=12.981055293868891}, {"VSignalRMS"=3.535562945845475, "VNoiseRMS"=0.00026784683978371324, "SNR(dB)"=82.41144093982854, "NumBits"=13.397249325552913, "SNRFS(dB)"=82.41136959658931, "NumBitsFS"=13.397237474516496}, {"VSignalRMS"=3.5355536437892874, "VNoiseRMS"=0.00017829890052506833, "SNR(dB)"=85.94617531834949, "NumBits"=13.984414504709218, "SNRFS(dB)"=85.9461268276916, "NumBitsFS"=13.984406449782657}, {"VSignalRMS"=3.535567447651429, "VNoiseRMS"=0.00014515019978032114, "SNR(dB)"=87.73282977463487, "NumBits"=14.281200959241673, "SNRFS(dB)"=87.73274737172412, "NumBitsFS"=14.281187271050518}] {"SNRFS(dB)" format="%_3p"; "NumBitsFS" format="%.1f"; "NumBits" format="%.1f"; "SNR(dB)" format="%_3p"; "VNoiseRMS" format="%#_3p"; "VSignalRMS" format="%#_3p"}
  out "Expected: Octaves 2-8":T1[](array[typedef])=[{"VSignalRMS"=3.5355339059327373, "VNoiseRMS"=0.0019933998557805812, "SNR(dB)"=64.97721167999286, "NumBits"=10.501197953487187, "SNRFS(dB)"=64.97721167999286, "NumBitsFS"=10.501197953487187}, {"VSignalRMS"=3.5355339059327373, "VNoiseRMS"=0.001409546555638735, "SNR(dB)"=67.98751163663268, "NumBits"=11.001247780171541, "SNRFS(dB)"=67.98751163663268, "NumBitsFS"=11.001247780171541}, {"VSignalRMS"=3.5355339059327373, "VNoiseRMS"=0.0009966999278902906, "SNR(dB)"=70.99781159327249, "NumBits"=11.501297606855895, "SNRFS(dB)"=70.99781159327249, "NumBitsFS"=11.501297606855895}, {"VSignalRMS"=3.5355339059327373, "VNoiseRMS"=0.0007047732778193675, "SNR(dB)"=74.0081115499123, "NumBits"=12.00134743354025, "SNRFS(dB)"=74.0081115499123, "NumBitsFS"=12.00134743354025}, {"VSignalRMS"=3.5355339059327373, "VNoiseRMS"=0.0004983499639451453, "SNR(dB)"=77.01841150655211, "NumBits"=12.501397260224604, "SNRFS(dB)"=77.01841150655211, "NumBitsFS"=12.501397260224604}, {"VSignalRMS"=3.5355339059327373, "VNoiseRMS"=0.00035238663890968373, "SNR(dB)"=80.02871146319193, "NumBits"=13.001447086908957, "SNRFS(dB)"=80.02871146319193, "NumBitsFS"=13.001447086908957}, {"VSignalRMS"=3.5355339059327373, "VNoiseRMS"=0.00024917498197257266, "SNR(dB)"=83.03901141983174, "NumBits"=13.501496913593312, "SNRFS(dB)"=83.03901141983174, "NumBitsFS"=13.501496913593312}, {"VSignalRMS"=3.5355339059327373, "VNoiseRMS"=0.00017619331945484186, "SNR(dB)"=86.04931137647155, "NumBits"=14.001546740277666, "SNRFS(dB)"=86.04931137647155, "NumBitsFS"=14.001546740277666}, {"VSignalRMS"=3.5355339059327373, "VNoiseRMS"=0.00012458749098628633, "SNR(dB)"=89.05961133311136, "NumBits"=14.50159656696202, "SNRFS(dB)"=89.05961133311136, "NumBitsFS"=14.50159656696202}] {"SNRFS(dB)" format="%_3p"; "NumBitsFS" format="%.1f"; "NumBits" format="%.1f"; "SNR(dB)" format="%_3p"; "VNoiseRMS" format="%#_3p"; "VSignalRMS" format="%#_3p"}
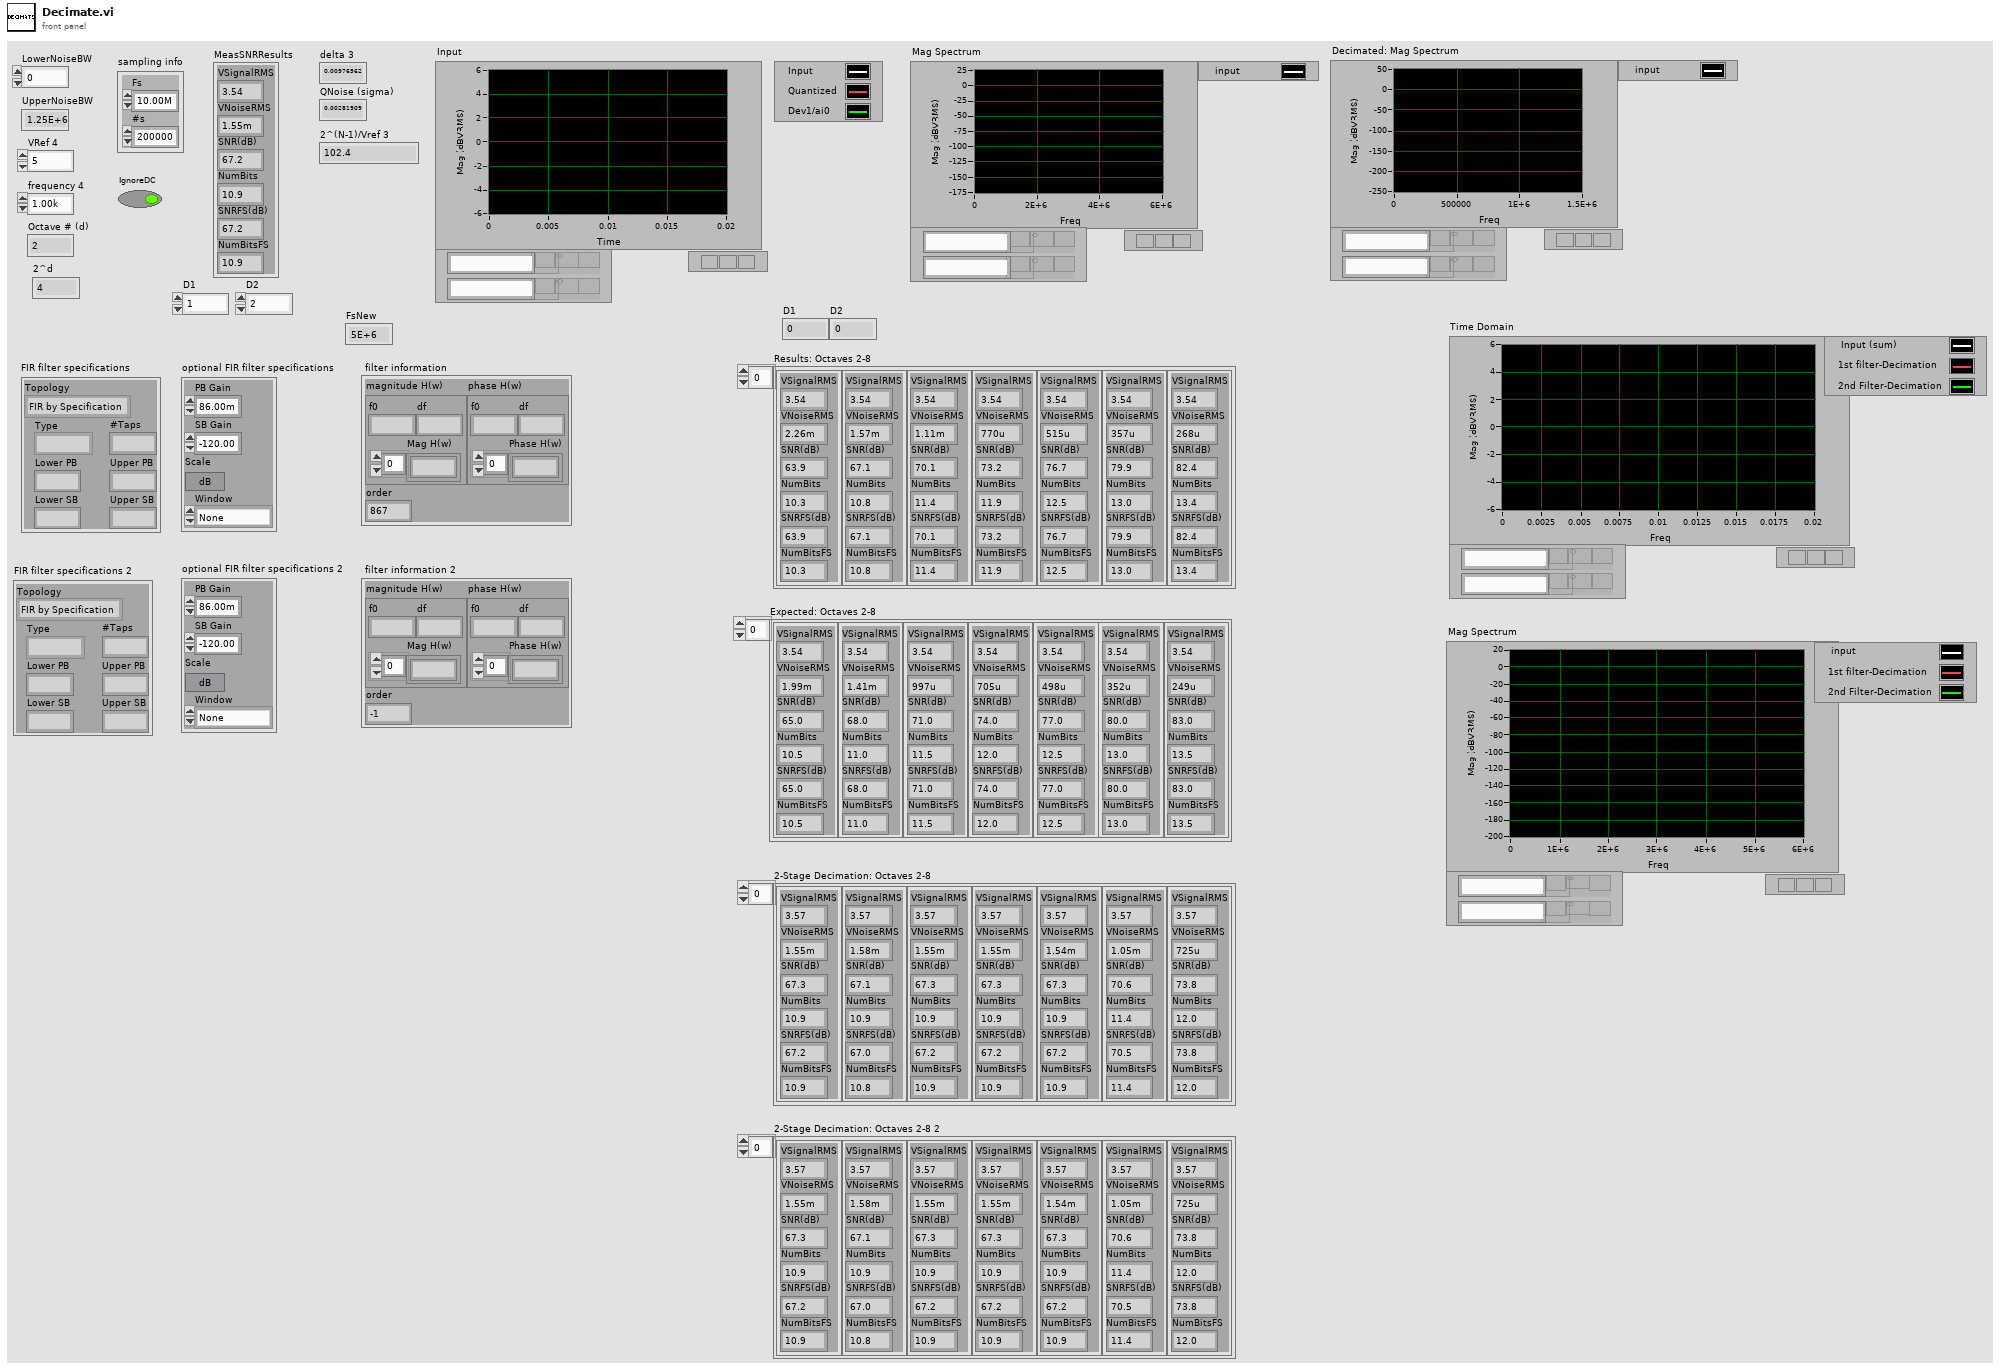
[diagram p1: front panel]
types:
  T1 = typedef "MeasSNRResults.ctl" = cluster{"VSignalRMS":dbl, "VNoiseRMS":dbl, "SNR(dB)":dbl, "NumBits":dbl, "SNRFS(dB)":dbl, "NumBitsFS":dbl}
  T2 = cluster{"Topology":enum16{"Off", "FIR by Specification", "Equi-ripple FIR", "Windowed FIR"}, "Type":enum16{"Lowpass", "Highpass", "Bandpass", "Bandstop"}, "#Taps":i32, "Lower PB":dbl, "Upper PB":dbl, "Lower SB":dbl, "Upper SB":dbl}
  T3 = cluster{"magnitude H(w)":cluster{"f0":dbl, "df":dbl, "Mag H(w)":dbl[]}, "phase H(w)":cluster{"f0":dbl, "df":dbl, "Phase H(w)":dbl[]}, "order":i32}
  T4 = cluster{"PB Gain":dbl, "SB Gain":dbl, "Scale":bool, "Window":enum16{"None", "Hanning", "Hamming", "Triangular", "Blackman", "Exact Blackman", "Blackman-Harris", "Kaiser-Bessel", "Flat Top"}}
  T5 = enum16{"Sine Wave", "Triangle Wave", "Square Wave", "Sawtooth Wave"}
  T6 = cluster{"averaging mode":u16, "weighting mode":u16, "number of averages":u32}
  T7 = cluster{"dB On (F)":bool, "unwrap phase (F)":bool, "convert to degree (F)":bool}
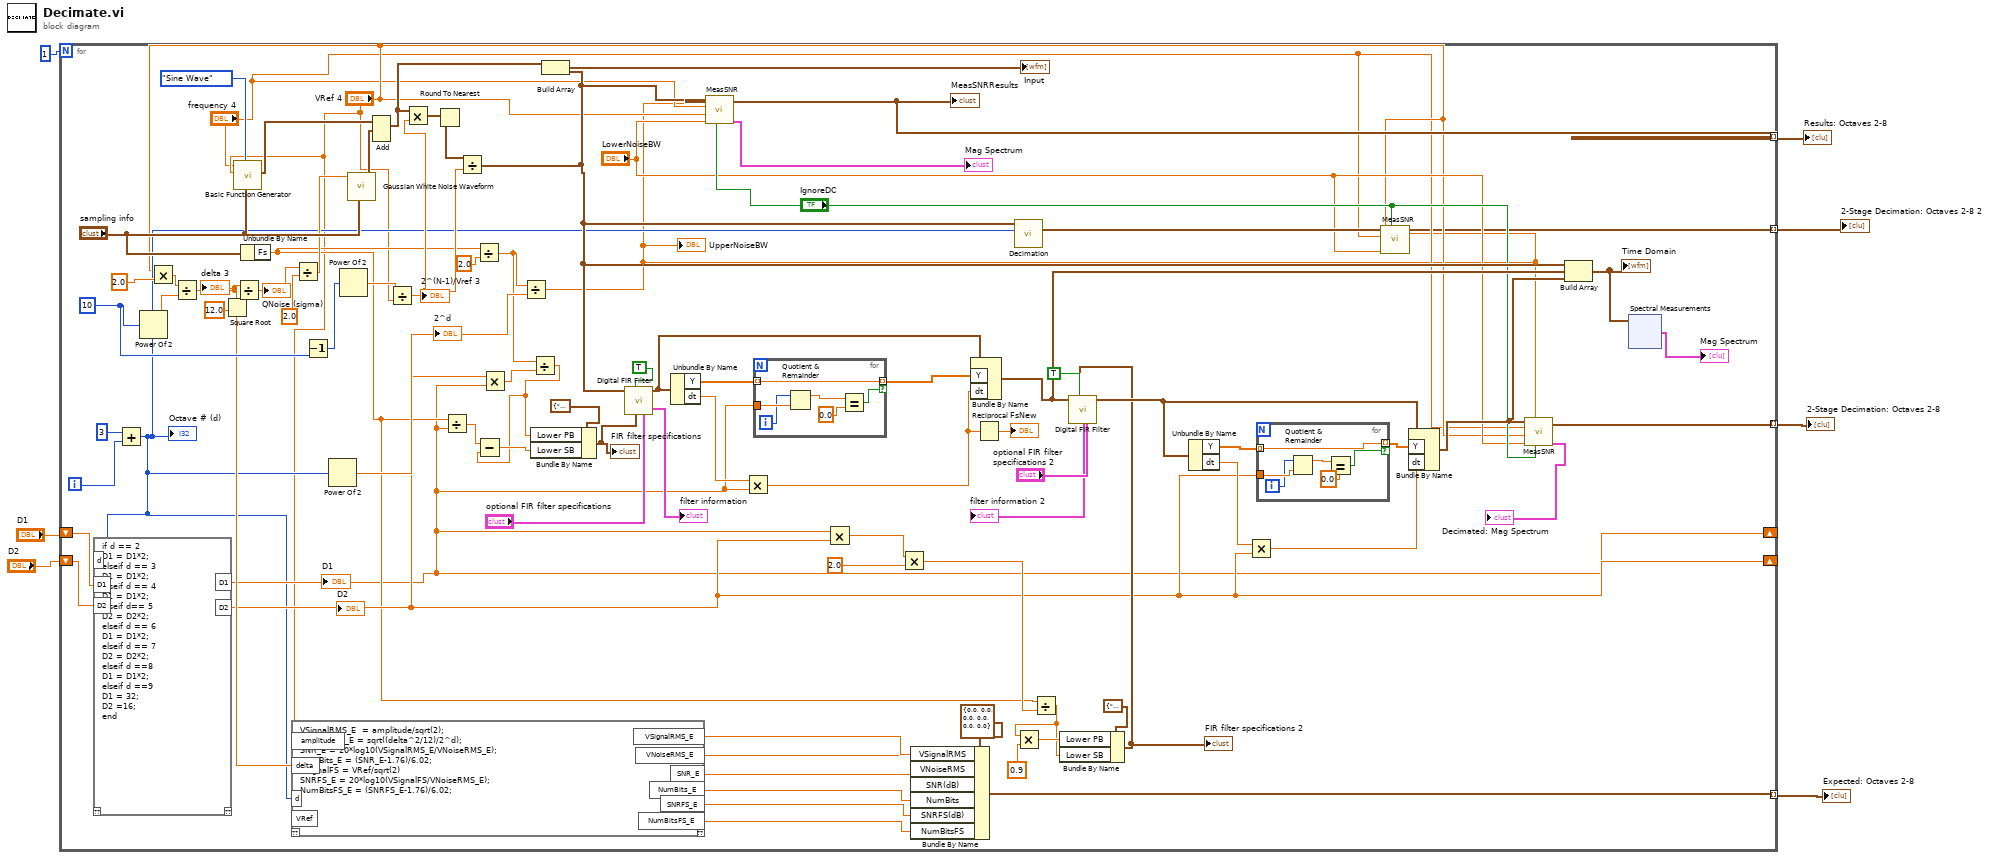
[diagram p0: block diagram]
diagram:
  n1 = for {
    N: 1 -> [_]
    tunnel: [w72] -> w7 mode=indexing
    tunnel: [w71] -> w6 mode=indexing
    tunnel: [w52] -> w4 mode=indexing
    shift-right: [w25] -> _
    shift-left: "D2" -> [w27]
    shift-right: [w23] -> _
    shift-left: "D1" -> [w26]
    tunnel: [w8] -> w1 mode=indexing
    i -> [w64]
    w70 = 10 ("x")
    n2 = Add(x=3, y=w64) -> (x+y=w15:i32)
    "Octave # (d)" <- w15
    n3 = mathscript code="if d == 2\nD1 = D1*2;\nelseif d == 3\nD1 = D1*2;\nelseif d == 4\nD1 = D1*2;\nelseif d== 5\nD2 = D2*2;\nelseif d == 6\nD1 = D1*2;\nelseif d == 7\nD2 = D2*2;\nelseif d ==8\nD1 = D1*2;\nelseif d ==9\nD1 = 32;\nD2 =16;\nend"("d"=w15, "D1"=w26, "D2"=w27) -> ("D1"=w23:dbl, "D2"=w25:dbl)  [unwired: 1 in, 1 out]
    "D1" <- w23
    "D2" <- w25
    n4 = Power Of 2(x=w70) -> (2^x=w93:dbl)
    n5 = Multiply(x="VRef 4", y=2.0) -> (x*y=w94:dbl)
    n6 = Divide(x=w94, y=w93) -> (x/y=w61:dbl)
    "delta 3" <- w61
    n7 = Square Root(x=12.0) -> (sqrt(x)=w92:dbl)
    n8 = call <vilib>:"Basic Function Generator.vi"("sampling info"="sampling info", "signal type"=T5."Sine Wave", "amplitude"="VRef 4", "frequency"="frequency 4") -> ("signal out"=w67:waveform(dbl))  [unwired: 5 in, 2 out]
    n9 = Divide(x=w61, y=w92) -> (x/y=w80:dbl)
    "QNoise (sigma)" <- w80
    n10 = Unbundle By Name("sampling info") -> ("Fs"=w24:dbl)
    n11 = mathscript code="VSignalRMS_E  = amplitude/sqrt(2);\nVNoiseRMS_E = sqrt((delta^2/12)/2^d);\nSNR_E = 20*log10(VSignalRMS_E/VNoiseRMS_E);\nNumBits_E = (SNR_E-1.76)/6.02;\nVSignalFS = VRef/sqrt(2)\nSNRFS_E = 20*log10(VSignalFS/VNoiseRMS_E);\nNumBitsFS_E = (SNRFS_E-1.76)/6.02;"("amplitude"="VRef 4", "VRef"="VRef 4", "d"=w15, "delta"=w61) -> ("VNoiseRMS_E"=w85:cdb, "SNR_E"=w84:cdb, "VSignalRMS_E"=w86:cdb, "NumBits_E"=w83:cdb, "SNRFS_E"=w82:cdb, "NumBitsFS_E"=w81:cdb)  [unwired: 1 in, 1 out]
    n12 = Divide(x=w80, y=2.0) -> (x/y=w68:dbl)
    n13 = Decrement(x=w70) -> (x-1=w91:i32)
    n14 = Power Of 2(x=w15) -> (2^x=w47:dbl)
    "2^d" <- w47
    n15 = Power Of 2(x=w91) -> (2^x=w87:dbl)
    n16 = call <vilib>:"Gaussian White Noise Waveform.vi"("sampling info"="sampling info", "standard deviation"=w68) -> ("signal out"=w66:waveform(dbl))  [unwired: 8 in, 1 out]
    n17 = Add(1:w66, 2:w67) -> (0:w65:waveform(dbl))  [unwired: 1 in, 1 out]
    n18 = Divide(x=w87, y="VRef 4") -> (x/y=w90:dbl)
    "2^(N-1)/Vref 3" <- w90
    n19 = Multiply(x=w65, y=w90) -> (x*y=w89:waveform(dbl))
    n20 = Round To Nearest(number=w89) -> (nearest integer value=w88:waveform(dbl))
    n21 = Divide(x=w24, y=w23) -> (x/y=w29:dbl)
    n22 = Divide(x=w88, y=w90) -> (x/y=w16:waveform(dbl))
    n23 = Divide(x=w24, y=2.0) -> (x/y=w32:dbl)
    n24 = Multiply(x=w25, y=w23) -> (x*y=w33:dbl)
    n25 = Divide(x=w32, y=w47) -> (x/y=w9:dbl)
    "UpperNoiseBW" <- w9
    n26 = Divide(x=w32, y=w33) -> (x/y=w22:dbl)
    n27 = Subtract(x=w29, y=w22) -> (x-y=w28:dbl)
    n28 = Bundle By Name(cluster=T2 {"Topology"=enum."FIR by Specification", "Type"=enum."Lowpass", "#Taps"=0, "Lower PB"=100.0, "Upper PB"=0.0, "Lower SB"=0.0, "Upper SB"=0.0} ("FIR filter specifications"), "Lower PB"=w22, "Lower SB"=w28) -> (w31:T2)
    "FIR filter specifications" <- w31
    n29 = Build Array(w65, w16) -> (→"Input":waveform(dbl)[])
    n30 = call-poly <vilib>:"Digital FIR Filter.vi"("optional FIR filter specifications"="optional FIR filter specifications", "FIR filter specifications"=w31, "reset filter"=TRUE, "signal in"=w16) -> ("filter information"=→"filter information":T3, "signal out"=w18:waveform(dbl))  [unwired: 5 in, 1 out]
    n31 = Unbundle By Name(w18) -> ("Y"=w45:dbl[], "dt"=w30:dbl)
    n32 = call "MeasSNR.vi"("IgnoreDC"="IgnoreDC", "UpperNoiseBW"=w9, "LowerNoiseBW"="LowerNoiseBW", "VRef"="VRef 4", "FSignal"="frequency 4", "Input"=w16) -> ("Mag Spectrum"=→"Mag Spectrum":cluster{"f0":dbl, "df":dbl, "magnitude":dbl[]}, "MeasSNRResults"=w71:T1)  [unwired: 4 in]
    "MeasSNRResults" <- w71
    n33 = Multiply(x=w30, y=w23) -> (x*y=w43:dbl)
    n34 = for {
      tunnel: w45 -> [w322] mode=indexing
      tunnel: [w322] -> w44 mode=indexing if=w324
      tunnel: w23 -> [w323]
      i -> [w321]
      n35 = Quotient & Remainder(x=w321, y=w323) -> (x-y*floor(x/y)=w326:dbl)  [unwired: 1 out]
      n36 = Equal?(x=w326, y=0.0) -> (x = y?=w324:bool)
    }
    n37 = Multiply(x=w23, y=w25) -> (x*y=w41:dbl)
    n38 = Multiply(x=w41, y=2.0) -> (x*y=w40:dbl)
    n39 = Bundle By Name(cluster=T1 {"VSignalRMS"=0.0, "VNoiseRMS"=0.0, "SNR(dB)"=0.0, "NumBits"=0.0, "SNRFS(dB)"=0.0, "NumBitsFS"=0.0} ("MeasSNRResults"), "VSignalRMS"=w86, "VNoiseRMS"=w85, "SNR(dB)"=w84, "NumBits"=w83, "SNRFS(dB)"=w82, "NumBitsFS"=w81) -> (w72:T1)
    n40 = Bundle By Name(cluster=w18, "Y"=w44, "dt"=w43) -> (w17:waveform(dbl))
    n41 = Reciprocal(x=w43) -> (1/x=→"FsNew":dbl)
    n42 = call "Decimation.vi"("d"=w15, "signal in"=w16) -> ("output waveform"=w14:waveform(dbl))  [unwired: 9 in]
    n43 = Divide(x=w24, y=w40) -> (x/y=w34:dbl)
    n44 = Multiply(x=w34, y=0.9) -> (x*y=w35:dbl)
    n45 = Bundle By Name(cluster=T2 {"Topology"=enum."FIR by Specification", "Type"=enum."Lowpass", "#Taps"=0, "Lower PB"=100.0, "Upper PB"=0.0, "Lower SB"=0.0, "Upper SB"=0.0} ("FIR filter specifications"), "Lower PB"=w35, "Lower SB"=w34) -> (w37:T2)
    "FIR filter specifications 2" <- w37
    n46 = call-poly <vilib>:"Digital FIR Filter.vi"("optional FIR filter specifications"="optional FIR filter specifications 2", "FIR filter specifications"=w37, "reset filter"=TRUE, "signal in"=w17) -> ("filter information"=→"filter information 2":T3, "signal out"=w53:waveform(dbl))  [unwired: 5 in, 1 out]
    n47 = Unbundle By Name(w53) -> ("Y"=w39:dbl[], "dt"=w54:dbl)
    n48 = Multiply(x=w54, y=w25) -> (x*y=w55:dbl)
    n49 = for {
      tunnel: [w316] -> w38 mode=indexing if=w318
      tunnel: w39 -> [w316] mode=indexing
      tunnel: w25 -> [w317]
      i -> [w315]
      n50 = Quotient & Remainder(x=w315, y=w317) -> (x-y*floor(x/y)=w320:dbl)  [unwired: 1 out]
      n51 = Equal?(x=w320, y=0.0) -> (x = y?=w318:bool)
    }
    n52 = call "MeasSNR.vi"("IgnoreDC"="IgnoreDC", "UpperNoiseBW"=w9, "LowerNoiseBW"="LowerNoiseBW", "VRef"="VRef 4", "FSignal"="frequency 4", "Input"=w14) -> ("MeasSNRResults"=w8:T1)  [unwired: 4 in, 1 out]
    n53 = Bundle By Name(cluster=w53, "Y"=w38, "dt"=w55) -> (w19:waveform(dbl))
    n54 = call "MeasSNR.vi"("IgnoreDC"="IgnoreDC", "UpperNoiseBW"=w9, "LowerNoiseBW"="LowerNoiseBW", "VRef"="VRef 4", "FSignal"="frequency 4", "Input"=w19) -> ("Mag Spectrum"=→"Decimated: Mag Spectrum":cluster{"f0":dbl, "df":dbl, "magnitude":dbl[]}, "MeasSNRResults"=w52:T1)  [unwired: 4 in]
    n55 = Build Array(w16, w17, w19) -> (w20:waveform(dbl)[])
    "Time Domain" <- w20
    n56 = xnode "Spectral Measurements"("Signals"=w20) -> ("FFT - (RMS)"=→"Mag Spectrum":cluster{"f0":dbl, "df":dbl, "magnitude":dbl[]}[])  [unwired: 1 in, 2 out]
  }
  "Expected: Octaves 2-8" <- w7
  "Results: Octaves 2-8" <- w6
  "2-Stage Decimation: Octaves 2-8" <- w4
  "2-Stage Decimation: Octaves 2-8 2" <- w1
